vi "TLB Native Dynamic Events ver 0.26a.vi"() -> ()   [LabVIEW 2018] (continued)
      tunnel: w241 -> [w2776 w2788 w2804 w2825 w2838 w2853 w2867 w2881 w2897 w2912 w2925 w2937 w2953 w2971 w2992 w3008 w3025 w3036 w3063 w3079 w3090 w3103 w3118 w3131 w3146 w3171 w3207 w3233 w3247 w3258 w3270 w3286 w3302 w3315 w3326 w3351 w3374 w3386 w3396 w3407 w3420 w3433 w3446 w3461 w3472 w3489 w3503 w3517 w3532 w3547 w3562 w3577 w3592 w3606]
      tunnel: [w2776 w2788 w2804 w2825 w2838 w2853 w2867 w2881 w2897 w2912 w2925 w2937 w2953 w2971 w2992 w3008 w3025 w3036 w3062 w3079 w3090 w3103 w3118 w3131 w3146 w3170 w3206 w3233 w3247 w3258 w3270 w3286 w3302 w3315 w3326 w3351 w3374 w3386 w3396 w3407 w3420 w3433 w3446 w3461 w3472 w3489 w3502 w3517 w3532 w3547 w3562 w3577 w3592 w3606] -> w240
      tunnel: w238 -> [w2775 w2787 w2802 w2826 w2836 w2851 w2865 w2880 w2895 w2910 w2924 w2936 w2952 w2964 w2987 w3009 w3026 w3035 w3053 w3078 w3089 w3102 w3117 w3130 w3145 w3167 w3203 w3232 w3244 w3257 w3269 w3285 w3301 w3314 w3325 w3352 w3375 w3387 w3395 w3406 w3417 w3430 w3443 w3462 w3473 w3490 w3497 w3518 w3533 w3548 w3563 w3578 w3593 w3607]
      tunnel: [w2775 w2787 w2802 w2826 w2836 w2851 w2865 w2880 w2895 w2910 w2924 w2936 w2952 w2964 w2986 w3009 w3026 w3035 w3052 w3078 w3089 w3102 w3117 w3130 w3145 w3166 w3202 w3232 w3244 w3257 w3269 w3285 w3301 w3314 w3325 w3352 w3375 w3387 w3395 w3406 w3417 w3430 w3443 w3462 w3473 w3490 w3497 w3518 w3533 w3548 w3563 w3578 w3593 w3607] -> w237
      tunnel: w235 -> [w2773 w2786 w2803 w2827 w2837 w2852 w2866 w2879 w2896 w2911 w2923 w2935 w2951 w2963 w2983 w3010 w3027 w3034 w3049 w3075 w3088 w3101 w3116 w3129 w3144 w3164 w3200 w3230 w3243 w3256 w3268 w3284 w3300 w3313 w3324 w3353 w3376 w3388 w3394 w3405 w3416 w3429 w3442 w3463 w3474 w3491 w3496 w3512 w3527 w3542 w3557 w3572 w3587 w3601]
      tunnel: [w2773 w2786 w2803 w2827 w2837 w2852 w2866 w2879 w2896 w2911 w2923 w2935 w2951 w2963 w2983 w3010 w3027 w3034 w3049 w3075 w3088 w3101 w3116 w3129 w3143 w3163 w3199 w3230 w3243 w3256 w3268 w3284 w3300 w3313 w3324 w3353 w3376 w3388 w3394 w3405 w3416 w3429 w3442 w3463 w3474 w3491 w3496 w3512 w3525 w3540 w3555 w3570 w3585 w3600] -> w234
      tunnel: w232 -> [_ _ _ _ _ _ _ _ _ _ _ _ _ _ _ _ _ _ _ _ _ _ _ _ _ _ _ _ _ _ _ _ _ _ _ _ _ _ _ _ _ _ _ _ _ w3482 _ _ _ _ _ _ _ _]
      tunnel: [w2772 w2785 w2797 w2817 w2831 w2846 w2861 w2875 w2891 w2905 w2920 w2934 w2945 w2962 w2980 w3001 w3028 w3033 w3046 w3074 w3087 w3100 w3115 w3126 w3137 w3157 w3191 w3229 w3242 w3255 w3273 w3278 w3294 w3310 w3322 w3337 w3369 w3380 w3400 w3404 w3415 w3428 w3441 w3454 w3475 w3480 w3495 w3511 w3522 w3537 w3552 w3567 w3582 w3597] -> w228
      tunnel: w229 -> [w2772 w2785 w2797 w2817 w2831 w2846 w2861 w2875 w2891 w2905 w2920 w2934 w2945 w2962 w2980 w3002 w3028 w3033 w3046 w3074 w3087 w3100 w3115 w3126 w3137 w3158 w3192 w3229 w3242 w3255 w3273 w3278 w3294 w3310 w3322 w3337 w3369 w3380 w3400 w3404 w3415 w3428 w3441 w3454 w3475 w3480 w3495 w3511 w3522 w3537 w3552 w3567 w3582 w3597]
      tunnel: w226 -> [_ _ _ _ _ _ _ _ w2890 _ _ _ _ _ _ _ _ _ _ _ _ _ _ _ _ _ _ _ _ _ _ _ _ _ _ _ _ _ _ _ _ _ _ _ _ _ _ _ _ _ _ _ _ _]
      tunnel: w224 -> [w2771 w2784 w2796 w2811 w2830 w2845 w2860 w2874 w2888 w2904 w2919 w2933 w2944 w2961 w2979 w2997 w3021 w3032 w3044 w3073 w3086 w3099 w3114 w3125 w3140 w3160 w3195 w3228 w3241 w3254 w3265 w3277 w3293 w3309 w3321 w3334 w3368 w3379 w3391 w3403 w3414 w3427 w3440 w3453 w3466 w3479 w3494 w3510 w3521 w3536 w3551 w3566 w3581 w3596]
      tunnel: [w2771 w2784 w2796 w2811 w2830 w2845 w2860 w2874 w2888 w2904 w2919 w2933 w2944 w2961 w2979 w2997 w3020 w3032 w3044 w3073 w3086 w3099 w3114 w3125 w3139 w3159 w3194 w3228 w3241 w3254 w3265 w3277 w3293 w3309 w3321 w3334 w3368 w3379 w3391 w3403 w3414 w3427 w3440 w3453 w3466 w3479 w3494 w3510 w3521 w3536 w3551 w3566 w3581 w3596] -> w223
      tunnel: [_ _ _ _ _ _ _ _ _ _ _ _ _ _ _ _ _ _ _ _ _ _ _ _ _ _ _ _ _ _ _ _ _ _ _ w3333 w3363 _ _ _ _ _ _ _ _ _ _ _ _ _ _ _ _ _] -> w221
      tunnel: w219 -> [w2770 w2783 w2795 w2810 w2829 w2844 w2859 w2873 w2887 w2903 w2918 w2932 w2943 w2960 w2978 w2996 w3012 w3031 w3042 w3072 w3085 w3098 w3113 w3124 w3141 w3161 w3196 w3227 w3240 w3253 w3264 w3276 w3292 w3308 w3320 w3332 w3367 w3378 w3390 w3402 w3413 w3426 w3439 w3452 w3465 w3478 w3493 w3509 w3520 w3535 w3550 w3565 w3580 w3595]
      tunnel: [w2770 w2783 w2795 w2810 w2829 w2844 w2859 w2873 w2887 w2903 w2918 w2932 w2943 w2960 w2978 w2996 w3012 w3031 w3042 w3072 w3085 w3098 w3113 w3124 w3141 w3161 w3196 w3227 w3240 w3253 w3264 w3276 w3292 w3308 w3320 w3332 w3367 w3378 w3390 w3402 w3413 w3426 w3439 w3452 w3465 w3478 w3493 w3509 w3520 w3535 w3550 w3565 w3580 w3595] -> w218
      tunnel: w214 -> [w2769 w2782 w2794 w2809 w2828 w2843 w2858 w2872 w2886 w2902 w2917 w2931 w2942 w2959 w2977 w2993 w3011 w3030 w3041 w3071 w3084 w3097 w3112 w3123 w3136 w3154 w3189 w3226 w3239 w3252 w3263 w3275 w3291 w3307 w3319 w3331 w3361 w3377 w3389 w3401 w3412 w3425 w3438 w3451 w3464 w3477 w3492 w3508 w3519 w3534 w3549 w3564 w3579 w3594]
      tunnel: [w2769 w2782 w2794 w2809 w2828 w2843 w2858 w2872 w2886 w2902 w2917 w2931 w2942 w2959 w2977 w2993 w3011 w3030 w3041 w3071 w3084 w3097 w3112 w3123 w3136 w3154 w3189 w3226 w3239 w3252 w3263 w3275 w3291 w3307 w3319 w3331 w3354 w3377 w3389 w3401 w3412 w3425 w3438 w3451 w3464 w3477 w3492 w3508 w3519 w3534 w3549 w3564 w3579 w3594] -> w213
      frame "Exit" {
        # ">>State Logic  >>"
        # ">>> Time cluster >>>"
        # ">>> Yaw >>>"
        # ">>> Stepper position >>>"
        # ">>> Encoders >>>"
        # ">>> Object detection >>>"
        # ">>> Ultrasonic Sensors Detect >>>"
        n70 = call "Imaq Dispose"("All Images? (No)"=TRUE) -> ()  [unwired: 5 in, 1 out]
      }
      frame "----Movement States----" {
        # ">>State Logic  >>"
        # ">>> Time cluster >>>"
        # ">>> Yaw >>>"
        # ">>> Stepper position >>>"
        # ">>> Encoders >>>"
        # ">>> Object detection >>>"
        # ">>> Ultrasonic Sensors Detect >>>"
      }
      frame "FORWARD" {
        # ">>State Logic  >>"
        # ">>> Time cluster >>>"
        # ">>> Yaw >>>"
        # ">>> Stepper position >>>"
        # ">>> Encoders >>>"
        # ">>> Object detection >>>"
        # ">>> Ultrasonic Sensors Detect >>>"
        n71 = Unbundle By Name(w2802) -> ("Yaw"=w2798:dbl)
        n72 = call "MOTOR CONTROL WITH PID AE.vi"("Yaw"=w2798, "Speed"=50.0, "Direction"=MOTOR_CONTROL_WITH_PID_AE_DIRECTION_TYPE_DEF."y-axis movement", "AE Mode"=MOTOR_CONTROL_WITH_PID_AE_DATA_MODE_TYPE_DEF."Write to AE") -> ()  [unwired: 1 out]
      }
      frame "FORWARD - IR ASSIST" {
        # ">>State Logic  >>"
        # ">>> Time cluster >>>"
        # ">>> Yaw >>>"
        # ">>> Stepper position >>>"
        # ">>> Encoders >>>"
        # ">>> Object detection >>>"
        # ">>> Ultrasonic Sensors Detect >>>"
        n73 = Unbundle By Name(w2817) -> ("Left IR Sensor"=w2816:dbl)
        n74 = Subtract(x=w2816, y=15.0) -> (x-y=w2814:dbl)
        n75 = Multiply(x=w2814, y=0.25) -> (x*y=w2812:dbl)
        n76 = call "MOTOR CONTROL WITH PID AE.vi"("Yaw"=w2812, "Speed"=30.0, "Direction"=MOTOR_CONTROL_WITH_PID_AE_DIRECTION_TYPE_DEF."y-axis movement", "AE Mode"=MOTOR_CONTROL_WITH_PID_AE_DATA_MODE_TYPE_DEF."Write to AE") -> ()  [unwired: 1 out]
      }
      frame "LEFT" {
        # ">>State Logic  >>"
        # ">>> Time cluster >>>"
        # ">>> Yaw >>>"
        # ">>> Stepper position >>>"
        # ">>> Encoders >>>"
        # ">>> Object detection >>>"
        # ">>> Ultrasonic Sensors Detect >>>"
        n77 = Unbundle By Name(w2836) -> ("Yaw"=w2833:dbl)
        n78 = call "MOTOR CONTROL WITH PID AE.vi"("Yaw"=w2833, "Speed"=-20.0, "Direction"=MOTOR_CONTROL_WITH_PID_AE_DIRECTION_TYPE_DEF."x-axis movement", "AE Mode"=MOTOR_CONTROL_WITH_PID_AE_DATA_MODE_TYPE_DEF."Write to AE") -> ()  [unwired: 1 out]
      }
      frame "RIGHT" {
        # ">>> Time cluster >>>"
        # ">>> Yaw >>>"
        # ">>> Stepper position >>>"
        # ">>> Encoders >>>"
        # ">>> Object detection >>>"
        # ">>> Ultrasonic Sensors Detect >>>"
        n79 = Unbundle By Name(w2851) -> ("Yaw"=w2847:dbl)
        n80 = call "MOTOR CONTROL WITH PID AE.vi"("Yaw"=w2847, "Speed"=20.0, "Direction"=MOTOR_CONTROL_WITH_PID_AE_DIRECTION_TYPE_DEF."x-axis movement", "AE Mode"=MOTOR_CONTROL_WITH_PID_AE_DATA_MODE_TYPE_DEF."Write to AE") -> ()  [unwired: 1 out]
      }
      frame "R-ACW" {
        # ">>> IR Sensors >>>"
        # ">>> Time cluster >>>"
        # ">>> Yaw >>>"
        # ">>> Stepper position >>>"
        # ">>> Encoders >>>"
        # ">>> Object detection >>>"
        # ">>> Ultrasonic Sensors Detect >>>"
        n81 = call "MOTOR CONTROL WITH PID AE.vi"("Speed"=10.0, "Direction"=MOTOR_CONTROL_WITH_PID_AE_DIRECTION_TYPE_DEF."rotation", "AE Mode"=MOTOR_CONTROL_WITH_PID_AE_DATA_MODE_TYPE_DEF."Write to AE") -> ()  [unwired: 1 in, 1 out]
      }
      frame "R-CW" {
        (unwired) -0.2 ("Speed")
        # ">>> Time cluster >>>"
        # ">>> Yaw >>>"
        # ">>> Stepper position >>>"
        # ">>> Encoders >>>"
        # ">>> Object detection >>>"
        # ">>> Ultrasonic Sensors Detect >>>"
        n82 = call "MOTOR CONTROL WITH PID AE.vi"("Speed"=-10.0, "Direction"=MOTOR_CONTROL_WITH_PID_AE_DIRECTION_TYPE_DEF."rotation", "AE Mode"=MOTOR_CONTROL_WITH_PID_AE_DATA_MODE_TYPE_DEF."Write to AE") -> ()  [unwired: 1 in, 1 out]
      }
      frame "X AXIS - SLOW" {
        # ">>> Line Sensor Cluster>>>"
        # ">>> IR Sensors >>>"
        # ">>> Time cluster >>>"
        # ">>> Yaw >>>"
        # ">>> Stepper position >>>"
        # ">>> Encoders >>>"
        # ">>> Object detection >>>"
        # ">>> Ultrasonic Sensors Detect >>>"
        n83 = Unbundle By Name(w2890) -> ("xSpeed"=w2889:dbl)
        n84 = Unbundle By Name(w2895) -> ("Yaw"=w2892:dbl)
        n85 = call "MOTOR CONTROL WITH PID AE.vi"("Yaw"=w2892, "Speed"=w2889, "Direction"=MOTOR_CONTROL_WITH_PID_AE_DIRECTION_TYPE_DEF."x-axis movement", "AE Mode"=MOTOR_CONTROL_WITH_PID_AE_DATA_MODE_TYPE_DEF."Write to AE") -> ()  [unwired: 1 out]
      }
      frame "REVERSE" {
        # ">>> Time cluster >>>"
        # ">>> Yaw >>>"
        # ">>> Stepper position >>>"
        # ">>> Encoders >>>"
        # ">>> Object detection >>>"
        # ">>> Ultrasonic Sensors Detect >>>"
        n86 = Unbundle By Name(w2910) -> ("Yaw"=w2906:dbl)
        n87 = call "MOTOR CONTROL WITH PID AE.vi"("Yaw"=w2906, "Speed"=-50.0, "Direction"=MOTOR_CONTROL_WITH_PID_AE_DIRECTION_TYPE_DEF."y-axis movement", "AE Mode"=MOTOR_CONTROL_WITH_PID_AE_DATA_MODE_TYPE_DEF."Write to AE") -> ()  [unwired: 1 out]
      }
      frame "STOP" {
        n88 = Wait (ms)(milliseconds to wait=u32 100) -> ()  [unwired: 1 out]
        n89 = call "MOTOR CONTROL WITH PID AE.vi"("Direction"=MOTOR_CONTROL_WITH_PID_AE_DIRECTION_TYPE_DEF."stop", "AE Mode"=MOTOR_CONTROL_WITH_PID_AE_DATA_MODE_TYPE_DEF."Write to AE") -> ()  [unwired: 2 in, 1 out]
      }
      frame "----SENSOR READING---- " {
      }
      frame "READ ENCODERS" {
        # ">>> Time cluster >>>"
        # ">>> Yaw >>>"
        # ">>> Stepper position >>>"
        # ">>> Object detection >>>"
        # ">>> Current encoder distance >>>"
        # ">>> Ultrasonic Sensors Detect >>>"
        n90 = call "MOTOR CONTROL WITH PID AE.vi"("AE Mode"=MOTOR_CONTROL_WITH_PID_AE_DATA_MODE_TYPE_DEF."Read from AE") -> ("Speed & distance"=w2949:T15)  [unwired: 3 in]
        n91 = Unbundle By Name(w2949) -> ("xDistance"=w2948:dbl, "yDistance"=w2947:dbl, "wDistance"=w2946:dbl)
        n92 = Bundle By Name(cluster=w2956, "xDistance"=w2948, "yDistance"=w2947, "wDistance"=w2946) -> (w2955:T8)
      }
      frame "READ ULTRASONIC" {
        (unwired) navX_type_def."Read Values" ("Mode")
        (unwired) MOTOR_CONTROL_NO_PID_Type_Def."Latch" ("Direction")
        # ">>> Line Sensor Cluster>>>"
        # ">>> IR Sensors >>>"
        # ">>State Logic  >>"
        # ">>> Time cluster >>>"
        # ">>> Ultrasonic Sensors Detect >>>"
        # ">>> Object detection >>>"
        # ">>> Encoders >>>"
        # ">>> Stepper position >>>"
        # ">>> Yaw >>>"
        n93 = call "Arduino Interfacing VI.vi"("AE Mode"=Arduino_Interfacing."Read From Arduino") -> ("Arduino Data"=w2969:T17)  [unwired: 3 in, 1 out]
        n94 = Unbundle By Name(w2969) -> ("PING A"=w2968:u8, "PING B"=w2967:u8, "PING C"=w2966:u8, "PING D"=w2965:u8)
        n95 = Bundle By Name(cluster=w2975, "PING_A"=w2968, "PING_B"=w2967, "PING_C"=w2966, "PING_D"=w2965) -> (w2976:T9)
      }
      frame "READ NAVX" {
        # ">> Item Selection Bias >>"
        # ">>State Logic  >>"
        # ">>> Line Sensor Cluster>>>"
        # ">>> IR Sensors >>>"
        # ">>> Time cluster >>>"
        # ">>> Yaw >>>"
        # ">>> Ultrasonic Sensors Detect >>>"
        # ">>> Object detection >>>"
        # ">>> Encoders >>>"
        # ">>> Stepper position >>>"
        n96 = call "navX reading VI.vi"("Mode"=navX_type_def."Read Values") -> ("NavX Readings"=w2982:T16)  [unwired: 2 in, 3 out]
        n97 = Unbundle By Name(w2982) -> ("Heading"=w2981:dbl)
        n98 = Unbundle By Name(w2982) -> ("Yaw"=w2985:dbl)
        n99 = Bundle By Name(cluster=w2987, "Yaw"=w2985, "Compass"=w2981) -> (w2986:T6)
      }
      frame "READ IR" {
        w2995 = T41 [enum."B/AI2"] items=["Not Connected", "AudioIn/Left", "AudioIn/Right", "C/AI0", "C/AI1", "A/AI0", "A/AI1", "A/AI2", "A/AI3", "A/AI4", "A/AI5", "A/AI6", "A/AI7", "B/AI0", "B/AI1", "B/AI2", "B/AI3", "B/AI4", "B/AI5", "B/AI6", "B/AI7", "AI/AI0", "AI/AI1", "AI/AI2", "AI/AI3", "A/AI0 (DIFF)", "A/AI1 (DIFF)", "A/AI2 (DIFF)", "A/AI3 (DIFF)", "B/AI0 (DIFF)", "B/AI1 (DIFF)", "B/AI2 (DIFF)", "B/AI3 (DIFF)"] ("AI Channel")
        w2999 = T41 [enum."B/AI1"] items=["Not Connected", "AudioIn/Left", "AudioIn/Right", "C/AI0", "C/AI1", "A/AI0", "A/AI1", "A/AI2", "A/AI3", "A/AI4", "A/AI5", "A/AI6", "A/AI7", "B/AI0", "B/AI1", "B/AI2", "B/AI3", "B/AI4", "B/AI5", "B/AI6", "B/AI7", "AI/AI0", "AI/AI1", "AI/AI2", "AI/AI3", "A/AI0 (DIFF)", "A/AI1 (DIFF)", "A/AI2 (DIFF)", "A/AI3 (DIFF)", "B/AI0 (DIFF)", "B/AI1 (DIFF)", "B/AI2 (DIFF)", "B/AI3 (DIFF)"] ("AI Channel")
        w3004 = T41 [enum."B/AI0"] items=["Not Connected", "AudioIn/Left", "AudioIn/Right", "C/AI0", "C/AI1", "A/AI0", "A/AI1", "A/AI2", "A/AI3", "A/AI4", "A/AI5", "A/AI6", "A/AI7", "B/AI0", "B/AI1", "B/AI2", "B/AI3", "B/AI4", "B/AI5", "B/AI6", "B/AI7", "AI/AI0", "AI/AI1", "AI/AI2", "AI/AI3", "A/AI0 (DIFF)", "A/AI1 (DIFF)", "A/AI2 (DIFF)", "A/AI3 (DIFF)", "B/AI0 (DIFF)", "B/AI1 (DIFF)", "B/AI2 (DIFF)", "B/AI3 (DIFF)"] ("AI Channel")
        # ">>> Line Sensor Cluster>>>"
        # ">>> IR Sensors >>>"
        # ">>State Logic  >>"
        # ">>> Time cluster >>>"
        # ">>> Ultrasonic Sensors Detect >>>"
        # ">>> Object detection >>>"
        # ">>> Encoders >>>"
        # ">>> Stepper position >>>"
        # ">>> Yaw >>>"
        n100 = call <vilib>:"Sharp IR.vi"("AI Channel"=w3004) -> ("Sharp IR Distance"=w3000:dbl)  [unwired: 8 in, 2 out]
        n101 = call <vilib>:"Sharp IR.vi"("AI Channel"=w2999) -> ("Sharp IR Distance"=w2998:dbl)  [unwired: 8 in, 2 out]
        n102 = call <vilib>:"Sharp IR.vi"("AI Channel"=w2995) -> ("Sharp IR Distance"=w2994:dbl)  [unwired: 8 in, 2 out]
        n103 = Bundle By Name(cluster=w3002, "Left IR Sensor"=w3000, "Arm IR Sensor"=w2998, "Bottom IR Sensor"=w2994) -> (w3001:T5)
      }
      frame "READ LINE SENSOR" {
        # ">>> IR Sensors >>>"
        # ">>> Line Sensor Cluster>>>"
        # ">>State Logic  >>"
        # ">>> Time cluster >>>"
        # ">>> Object detection >>>"
        # ">>> Yaw >>>"
        # ">>> Ultrasonic Sensors Detect >>>"
        # ">>> Encoders >>>"
        # ">>> Stepper position >>>"
        n104 = call "Line Sensor AE.vi"("AE State"=Line_Sensor_AE_Type_Def."READ FROM LINE SENSORS") -> ("Line Detected?"=w3018:bool, "Line Sensor Raw Values"=w3017:T43)
        n105 = Unbundle By Name(w3017) -> ("S1"=w3016:dbl, "S2"=w3015:dbl, "S3"=w3014:dbl, "S4"=w3013:dbl)
        n106 = Bundle By Name(cluster=w3021, "Line Detected?"=w3018, "S1"=w3016, "S2"=w3015, "S3"=w3014, "S4"=w3013) -> (w3020:T4)
      }
      frame "----SYSTEM MODES----" {
        (unwired) I2C_MASTER_Type_Def."Last State" ("Arduino Mode")
        # ">>> Object detection >>>"
        # ">>> Yaw >>>"
        # ">>> Ultrasonic Sensors Detect >>>"
        # ">>> Encoders >>>"
        # ">>> Stepper position >>>"
      }
      frame "INIT" {
        w3064 = u8 0
        w3065 = 0.0
        # ">>> IR Sensors >>>"
        # ">>> IR Sensors >>>"
        # ">>> Line Sensor Cluster>>>"
        # ">>> Time cluster >>>"
        # ">>> Object detection >>>"
        # ">>> Yaw >>>"
        # ">>> Ultrasonic Sensors Detect >>>"
        # ">>> Encoders >>>"
        # ">>> Stepper position >>>"
        # ">>State Logic  >>"
        n107 = call "Arduino Interfacing VI.vi"("AE Mode"=Arduino_Interfacing."Initialize") -> ()  [unwired: 3 in, 2 out]
        n108 = call "FGV Stop.vi"("Init/Read/Write State"=States_for_Action_Engine."Initialize") -> ()  [unwired: 2 in, 2 out]
        n109 = call "Elasped Timer.vi"("Action"=Elapsed_timer_control."Initialize") -> ()  [unwired: 7 in, 4 out]
        n110 = call "MOTOR CONTROL WITH PID AE.vi"("AE Mode"=MOTOR_CONTROL_WITH_PID_AE_DATA_MODE_TYPE_DEF."Init AE") -> ()  [unwired: 3 in, 1 out]
        n111 = call "IMAQ Reference AE.vi"("IMAQ AE States"=IMAQ_Reference_AE."Initialize AE") -> ()  [unwired: 1 in, 2 out]
        n112 = call "Line Sensor AE.vi"("AE State"=Line_Sensor_AE_Type_Def."INIT AE") -> ()  [unwired: 2 out]
        n113 = Bundle By Name(cluster=w3058, "Recognized Object"=FALSE, "Object X coordinate"=0.0, "Object Y coordinate"=0.0) -> (w3057:T11)
        n114 = Bundle By Name(cluster=w3063, "y Stepper Position"=u8 0, "z Stepper Position"=u8 0) -> (w3062:T7)
        n115 = Bundle By Name(cluster=w3067, "xDistance"=w3065, "yDistance"=w3065, "wDistance"=w3065) -> (w3066:T8)
        n116 = Bundle By Name(cluster=w3069, "PING_A"=w3064, "PING_B"=w3064, "PING_C"=w3064, "PING_D"=w3064) -> (w3070:T9)
        n117 = Bundle By Name(cluster=w3053, "Yaw"=0.0) -> (w3052:T6)
      }
      frame "ARDUINO - ULTRASONIC" {
        # ">>> Time cluster >>>"
        # ">>> Line Sensor Cluster>>>"
        # ">>> Object detection >>>"
        # ">>> Yaw >>>"
        # ">>> Ultrasonic Sensors Detect >>>"
        # ">>> Encoders >>>"
        # ">>> Stepper position >>>"
        # ">>State Logic  >>"
        n118 = call "Arduino Interfacing VI.vi"("Data to Write"=I2C_MASTER_WRITE_NEW_Type_Def."Ultrasonic sensors", "AE Mode"=Arduino_Interfacing."Write to Arduino") -> ()  [unwired: 2 in, 2 out]
      }
      frame "NAVX CALIBRATE" {
        # ">>> Object detection >>>"
        # ">>> Yaw >>>"
        # ">>> Ultrasonic Sensors Detect >>>"
        # ">>> Encoders >>>"
        # ">>> Stepper position >>>"
        # ">>State Logic  >>"
        # "Adds a 15 second delay to the startup process \nfor the NavX to calibrate"
        n119 = Wait (ms)(milliseconds to wait=u32 1000) -> ()  [unwired: 1 out]
      }
      frame "NO ACTION", Default {
        (unwired) u8 0 ("y Stepper value")
        (unwired) TRUE ("Latch")
        (unwired) navX_type_def."Read Values" ("Mode")
        (unwired) MOTOR_CONTROL_NO_PID_Type_Def."Latch" ("Direction")
        # ">>> Object detection >>>"
        # ">>> Yaw >>>"
        # ">>> Ultrasonic Sensors Detect >>>"
        # ">>> Encoders >>>"
        # ">>> Stepper position >>>"
        # ">>State Logic  >>"
        n120 = case shown="4" w3106 {
          tunnel: [0 100] -> w3108
          frame 1, Default {
          }
          frame 4 {
          }
        }
      }
      frame "----RESET CASES----" {
        (unwired) I2C_MASTER_Type_Def."Last State" ("Arduino Mode")
        # ">>> Object detection >>>"
        # ">>> Yaw >>>"
        # ">>> Ultrasonic Sensors Detect >>>"
        # ">>> Encoders >>>"
        # ">>> Stepper position >>>"
        # ">>State Logic  >>"
      }
      frame "RESET ENCODERS" {
        # ">>> Object detection >>>"
        # ">>> Yaw >>>"
        # ">>> Ultrasonic Sensors Detect >>>"
        # ">>> Encoders >>>"
        # ">>> Stepper position >>>"
        # ">>State Logic  >>"
        n121 = call "MOTOR CONTROL WITH PID AE.vi"("Direction"=MOTOR_CONTROL_WITH_PID_AE_DIRECTION_TYPE_DEF."reset encoders", "AE Mode"=MOTOR_CONTROL_WITH_PID_AE_DATA_MODE_TYPE_DEF."Write to AE") -> ()  [unwired: 2 in, 1 out]
      }
      frame "RESET FLAGS" {
        # ">>> Line Sensor Cluster>>>"
        # ">>> IR Sensors >>>"
        # ">>> Time cluster >>>"
        # ">>> Object detection >>>"
        # ">>> Yaw >>>"
        # ">>> Ultrasonic Sensors Detect >>>"
        # ">>> Encoders >>>"
        # ">>> Stepper position >>>"
        # ">>> Line Sensor Cluster>>>"
        # ">>> IR Sensors >>>"
        # ">>> Time cluster >>>"
        # ">>> Object detection >>>"
        # ">>> Yaw >>>"
        # ">>> Ultrasonic Sensors Detect >>>"
        # ">>> Encoders >>>"
        # ">>> Stepper position >>>"
        # "Resets BOOLEAN FLAGS only"
        n122 = Wait (ms)(milliseconds to wait=u32 20) -> ()  [unwired: 1 out]
        n123 = Bundle By Name(cluster=w3150, "Recognized Object"=FALSE) -> (w3149:T11)
        n124 = Bundle By Name(cluster=w3140, "Line Detected?"=FALSE) -> (w3139:T4)
        n125 = Bundle By Name(cluster=w3144, "Time up flag"=FALSE) -> (w3143:T3)
      }
      frame "RESET SENSOR VALUES" {
        w3155 = 0.0 ("S4")
        w3156 = 0.0 ("S4")
        # "Resets SENSOR VALUES only"
        # ">>> Line Sensor Cluster>>>"
        # ">>> IR Sensors >>>"
        # ">>> Time cluster >>>"
        # ">>> Object detection >>>"
        # ">>> Yaw >>>"
        # ">>> Ultrasonic Sensors Detect >>>"
        # ">>> Encoders >>>"
        # ">>> Stepper position >>>"
        # ">>> Line Sensor Cluster>>>"
        # ">>> IR Sensors >>>"
        # ">>> Time cluster >>>"
        # ">>> Object detection >>>"
        # ">>> Yaw >>>"
        # ">>> Ultrasonic Sensors Detect >>>"
        # ">>> Encoders >>>"
        # ">>> Stepper position >>>"
        # "Resets any software variables\nand/or non-critical states"
        n126 = Wait (ms)(milliseconds to wait=u32 20) -> ()  [unwired: 1 out]
        n127 = Bundle By Name(cluster=w3164, "SET TIME TO CHECK"=0.0) -> (w3163:T3)
        n128 = Bundle By Name(cluster=w3180, "Object X coordinate"=0.0, "Object Y coordinate"=0.0) -> (w3179:T11)
        n129 = Bundle By Name(cluster=w3171, "y Stepper Position"=u8 0, "z Stepper Position"=u8 0) -> (w3170:T7)
        n130 = Bundle By Name(cluster=w3158, "Left IR Sensor"=w3155, "Arm IR Sensor"=w3155) -> (w3157:T5)
        n131 = Bundle By Name(cluster=w3176, "xDistance"=0.0, "yDistance"=0.0, "wDistance"=0.0) -> (w3175:T8)
        n132 = Bundle By Name(cluster=w3187, "PING_A"=u8 0, "PING_B"=u8 0, "PING_C"=u8 0, "PING_D"=u8 0) -> (w3186:T9)
        n133 = Bundle By Name(cluster=w3167, "Yaw"=0.0) -> (w3166:T6)
        n134 = Bundle By Name(cluster=w3160, "S1"=w3156, "S2"=w3156, "S3"=w3156, "S4"=w3156) -> (w3159:T4)
      }
      frame "RESET ALL SENSORS" {
        w3190 = 0.0 ("SET TIME TO CHECK")
        # ">>> Line Sensor Cluster>>>"
        # ">>> IR Sensors >>>"
        # ">>> Time cluster >>>"
        # ">>> Object detection >>>"
        # ">>> Yaw >>>"
        # ">>> Ultrasonic Sensors Detect >>>"
        # ">>> Encoders >>>"
        # ">>> Stepper position >>>"
        # ">>> Line Sensor Cluster>>>"
        # ">>> IR Sensors >>>"
        # ">>> Time cluster >>>"
        # ">>> Object detection >>>"
        # ">>> Yaw >>>"
        # ">>> Ultrasonic Sensors Detect >>>"
        # ">>> Encoders >>>"
        # ">>> Stepper position >>>"
        # "Resets ALL SENSOR PARAMTERS"
        n135 = Wait (ms)(milliseconds to wait=u32 20) -> ()  [unwired: 1 out]
        n136 = Bundle By Name(cluster=w3200, "Time up flag"=FALSE, "SET TIME TO CHECK"=0.0) -> (w3199:T3)
        n137 = Bundle By Name(cluster=w3217, "Recognized Object"=FALSE, "Object X coordinate"=0.0, "Object Y coordinate"=0.0) -> (w3216:T11)
        n138 = Bundle By Name(cluster=w3207, "y Stepper Position"=u8 0, "z Stepper Position"=u8 0) -> (w3206:T7)
        n139 = Bundle By Name(cluster=w3195, "Line Detected?"=FALSE) -> (w3194:T4)
        n140 = Bundle By Name(cluster=w3192, "Left IR Sensor"=w3190, "Arm IR Sensor"=w3190) -> (w3191:T5)
        n141 = Bundle By Name(cluster=w3212, "xDistance"=0.0, "yDistance"=0.0, "wDistance"=0.0) -> (w3211:T8)
        n142 = Bundle By Name(cluster=w3224, "PING_A"=u8 0, "PING_B"=u8 0, "PING_C"=u8 0, "PING_D"=u8 0) -> (w3223:T9)
        n143 = Bundle By Name(cluster=w3203, "Yaw"=0.0) -> (w3202:T6)
      }
      frame "RESET YAW" {
        n144 = Wait (ms)(milliseconds to wait=u32 100) -> ()  [unwired: 1 out]
        n145 = call "navX reading VI.vi"("Mode"=navX_type_def."Zero Yaw") -> ()  [unwired: 2 in, 4 out]
      }
      frame "RESET ARM" {
        n146 = call "Arduino Interfacing VI.vi"("Data to Write"=I2C_MASTER_WRITE_NEW_Type_Def."Soft Reset", "AE Mode"=Arduino_Interfacing."Write to Arduino") -> ()  [unwired: 2 in, 2 out]
      }
      frame "--------CAM STATES-------" {
      }
      frame "OPEN IMAQ REF" {
        # ">>> Line Sensor Cluster>>>"
        # ">>State Logic  >>"
        # ">>> Time cluster >>>"
        # ">>> Object detection >>>"
        # ">>> Yaw >>>"
        # ">>> Ultrasonic Sensors Detect >>>"
        # ">>> Encoders >>>"
        # ">>> Stepper position >>>"
        # ">>> IR Sensors >>>"
        n147 = call "IMAQ Reference AE.vi"("IMAQ AE States"=IMAQ_Reference_AE."Initialize AE") -> ()  [unwired: 1 in, 2 out]
      }
      frame "OPEN LOG CAM" {
        n148 = call "Webcam AE.vi"("Session In"=T39 "cam0", "Camera states"=Webcam_AE."Initialize Camera") -> ("error out"=w3281:errorcluster, "Session Out"=w3280:T39)  [unwired: 1 in, 1 out]
        n149 = call "Webcam AE.vi"("error in (no error)"=w3281, "Session In"=w3280, "Camera states"=Webcam_AE."Open Camera") -> ()  [unwired: 3 out]
      }
      frame "OPEN LIFE CAM" {
        n150 = call "Webcam AE.vi"("Session In"=T39 "cam1", "Camera states"=Webcam_AE."Initialize Camera") -> ("error out"=w3297:errorcluster, "Session Out"=w3296:T39)  [unwired: 1 in, 1 out]
        n151 = call "Webcam AE.vi"("error in (no error)"=w3297, "Session In"=w3296, "Camera states"=Webcam_AE."Open Camera") -> ()  [unwired: 3 out]
      }
      frame "CAM ACQ" {
        # ">>State Logic  >>"
        # ">>> Time cluster >>>"
        # ">>> Yaw >>>"
        # ">>> Stepper position >>>"
        # ">>> Encoders >>>"
        # ">>> Object detection >>>"
        # ">>> Ultrasonic Sensors Detect >>>"
        n152 = call "Webcam AE.vi"("Camera states"=Webcam_AE."Continuous Acquisition") -> ()  [unwired: 2 in, 3 out]
      }
      frame "CAM CLOSE" {
        # ">>State Logic  >>"
        # ">>> Time cluster >>>"
        # ">>> Yaw >>>"
        # ">>> Stepper position >>>"
        # ">>> Encoders >>>"
        # ">>> Object detection >>>"
        # ">>> Ultrasonic Sensors Detect >>>"
        n153 = call "Webcam AE.vi"("Camera states"=Webcam_AE."Close Camera") -> ()  [unwired: 2 in, 3 out]
      }
      frame "PROCESS IMAGE" {
        # ">>> Line Sensor Cluster>>>"
        # ">>> IR Sensors >>>"
        # ">> Item Selection Bias >>"
        # ">> Item Selection Bias >>"
        # ">>State Logic  >>"
        # ">>> Time cluster >>>"
        # ">>> Yaw >>>"
        # ">>> Stepper position >>>"
        # ">>> Encoders >>>"
        # ">>> Object detection >>>"
        # ">>> Ultrasonic Sensors Detect >>>"
        n154 = call "Webcam AE.vi"("Camera states"=Webcam_AE."Retrieve Image") -> ("error out"=w3345:errorcluster, "Image Out"=w3346:T45)  [unwired: 2 in, 1 out]
        n155 = call "IMAQ Reference AE.vi"("IMAQ AE States"=IMAQ_Reference_AE."Get IMAQ Reference") -> ("Image Out"=w3335:T45)  [unwired: 1 in, 1 out]
        n156 = call "Object Detection SubVI.vi"("Error In"=w3345, "Mode"=w3332, "Image Dest"=w3335, "Image in"=w3346) -> ("Error out"=w3333:errorcluster, "Object Center Coordinates"=w3342:cluster{"x":sgl, "y":sgl}, "Object detection cluster"=w3338:T46)  [unwired: 1 out]
        n157 = Unbundle By Name(w3338) -> ("Object detected?"=w3339:bool)
        n158 = Unbundle By Name(w3342) -> ("x"=w3341:sgl, "y"=w3340:sgl)
        n159 = Bundle By Name(cluster=w3344, "Recognized Object"=w3339, "Object X coordinate"=w3341, "Object Y coordinate"=w3340) -> (w3343:T11)
      }
      frame "COLOUR PROCESSING" {
        # ">>> Box Colour Detection >>>"
        # ">>> Box Colour Detection >>>"
        # ">>> Line Sensor Cluster>>>"
        # ">>> IR Sensors >>>"
        # ">> Item Selection Bias >>"
        # ">> Item Selection Bias >>"
        # ">>State Logic  >>"
        # ">>> Time cluster >>>"
        # ">>> Yaw >>>"
        # ">>> Stepper position >>>"
        # ">>> Encoders >>>"
        # ">>> Object detection >>>"
        # ">>> Ultrasonic Sensors Detect >>>"
        n160 = call "Webcam AE.vi"("Camera states"=Webcam_AE."Retrieve Image") -> ("error out"=w3364:errorcluster, "Image Out"=w3365:T45)  [unwired: 2 in, 1 out]
        n161 = call "Box Colour Detection SubVI.vi"("Image In"=w3365, "Error In"=w3364) -> ("Colour output boolean cluster"=w3362:T47, "Error out"=w3363:errorcluster)  [unwired: 1 out]
        n162 = Unbundle By Name(w3362) -> ("Red"=w3360:bool, "Black"=w3359:bool, "Blue"=w3358:bool, "Yellow"=w3357:bool, "Green"=w3356:bool, "No recognizable coolour"=w3355:bool)
        n163 = Bundle By Name(cluster=w3361, "Red"=w3360, "Black"=w3359, "Blue"=w3358, "Yellow"=w3357, "Green"=w3356, "Unknown"=w3355) -> (w3354:T1)
      }
      frame "DISPOSE CAM BUFFERS" {
        # ">> Item Selection Bias >>"
        # ">>> Line Sensor Cluster>>>"
        # ">>> IR Sensors >>>"
        # ">>State Logic  >>"
        # ">>> Time cluster >>>"
        # ">>> Yaw >>>"
        # ">>> Stepper position >>>"
        # ">>> Encoders >>>"
        # ">>> Object detection >>>"
        # ">>> Ultrasonic Sensors Detect >>>"
        n164 = call "Webcam AE.vi"("Camera states"=Webcam_AE."Dispose Camera Image Buffer") -> ()  [unwired: 2 in, 3 out]
      }
      frame "DISPOSE PROC BUFFERS" {
        # ">>> Line Sensor Cluster>>>"
        # ">>State Logic  >>"
        # ">>> IR Sensors >>>"
        # ">>> Time cluster >>>"
        # ">>> Object detection >>>"
        # ">>> Yaw >>>"
        # ">>> Ultrasonic Sensors Detect >>>"
        # ">>> Encoders >>>"
        # ">>> Stepper position >>>"
        n165 = call "IMAQ Reference AE.vi"("IMAQ AE States"=IMAQ_Reference_AE."Dispose Processing Buffer") -> ()  [unwired: 1 in, 2 out]
      }
      frame "-----ARM ACTIONS-----" {
      }
      frame "CLOSE CLAW" {
        n166 = call "Arduino Interfacing VI.vi"("Data to Write"=I2C_MASTER_WRITE_NEW_Type_Def."Close Claw", "AE Mode"=Arduino_Interfacing."Write to Arduino") -> ()  [unwired: 2 in, 2 out]
      }
      frame "OPEN CLAW" {
        n167 = call "Arduino Interfacing VI.vi"("Data to Write"=I2C_MASTER_WRITE_NEW_Type_Def."Open Claw", "AE Mode"=Arduino_Interfacing."Write to Arduino") -> ()  [unwired: 2 in, 2 out]
      }
      frame "Z STEPPER CAM HEIGHT" {
        n168 = call "Arduino Interfacing VI.vi"("Data to Write"=I2C_MASTER_WRITE_NEW_Type_Def."zStepper 6k", "AE Mode"=Arduino_Interfacing."Write to Arduino") -> ()  [unwired: 2 in, 2 out]
      }
      frame "Z STEPPER GRAB HEIGHT" {
        # ">>State Logic  >>"
        # ">>> Time cluster >>>"
        # ">>> Yaw >>>"
        # ">>> Stepper position >>>"
        # ">>> Encoders >>>"
        # ">>> Object detection >>>"
        # ">>> Ultrasonic Sensors Detect >>>"
        n169 = call "Arduino Interfacing VI.vi"("Data to Write"=I2C_MASTER_WRITE_NEW_Type_Def."zStepper 100", "AE Mode"=Arduino_Interfacing."Write to Arduino") -> ()  [unwired: 2 in, 2 out]
      }
      frame "Z STEPPER BOX HEIGHT" {
        # ">>> IR Sensors >>>"
        # ">>> Time cluster >>>"
        # ">>> Yaw >>>"
        # ">>> Stepper position >>>"
        # ">>> Encoders >>>"
        # ">>> Object detection >>>"
        # ">>> Ultrasonic Sensors Detect >>>"
        n170 = call "Arduino Interfacing VI.vi"("Data to Write"=I2C_MASTER_WRITE_NEW_Type_Def."zStepper 5k", "AE Mode"=Arduino_Interfacing."Write to Arduino") -> ()  [unwired: 2 in, 2 out]
      }
      frame "Y STEPPER CONTROL" {
        # ">>State Logic  >>"
        # ">>> yStepper command>>>"
        # ">>> Time cluster >>>"
        # ">>> Yaw >>>"
        # ">>> Stepper position >>>"
        # ">>> Encoders >>>"
        # ">>> Object detection >>>"
        # ">>> Ultrasonic Sensors Detect >>>"
        n171 = Unbundle By Name(w3482) -> ("yStepper desired"=w3481:u8)
        n172 = call "Arduino Interfacing VI.vi"("y Stepper value"=w3481, "Data to Write"=I2C_MASTER_WRITE_NEW_Type_Def."yStepper control", "AE Mode"=Arduino_Interfacing."Write to Arduino") -> ()  [unwired: 1 in, 2 out]
      }
      frame "READ STEPPER VALUES" {
        # ">>State Logic  >>"
        # ">>> Time cluster >>>"
        # ">>> Yaw >>>"
        # ">>> Stepper position >>>"
        # ">>> Encoders >>>"
        # ">>> Object detection >>>"
        # ">>> Ultrasonic Sensors Detect >>>"
        n173 = call "Arduino Interfacing VI.vi"("AE Mode"=Arduino_Interfacing."Read From Arduino") -> ("Arduino Data"=w3500:T17)  [unwired: 3 in, 1 out]
        n174 = Unbundle By Name(w3500) -> ("y Stepper Position"=w3499:u8, "z Stepper Position"=w3498:u8)
        n175 = Bundle By Name(cluster=w3503, "y Stepper Position"=w3499, "z Stepper Position"=w3498) -> (w3502:T7)
      }
      frame " -----TIMING-----" {
        # ">>State Logic  >>"
        # ">>> Time cluster >>>"
        # ">>> Yaw >>>"
        # ">>> Stepper position >>>"
        # ">>> Encoders >>>"
        # ">>> Object detection >>>"
        # ">>> Ultrasonic Sensors Detect >>>"
      }
      frame "SET TIMER 1" {
        # ">>State Logic  >>"
        # ">>> Time cluster >>>"
        # ">>> Yaw >>>"
        # ">>> Stepper position >>>"
        # ">>> Encoders >>>"
        # ">>> Object detection >>>"
        # ">>> Ultrasonic Sensors Detect >>>"
        n176 = call "Elasped Timer.vi"("Time Setting"=1.0, "Action"=Elapsed_timer_control."Initialize") -> ()  [unwired: 6 in, 4 out]
        n177 = Bundle By Name(cluster=w3527, "Time up flag"=FALSE) -> (w3525:T3)
      }
      frame "SET TIMER 2" {
        # ">>State Logic  >>"
        # ">>> Time cluster >>>"
        # ">>> Yaw >>>"
        # ">>> Stepper position >>>"
        # ">>> Encoders >>>"
        # ">>> Object detection >>>"
        # ">>> Ultrasonic Sensors Detect >>>"
        n178 = call "Elasped Timer.vi"("Time Setting"=2.0, "Action"=Elapsed_timer_control."Initialize") -> ()  [unwired: 6 in, 4 out]
        n179 = Bundle By Name(cluster=w3542, "Time up flag"=FALSE) -> (w3540:T3)
      }
      frame "SET TIMER 3" {
        # ">>State Logic  >>"
        # ">>> Time cluster >>>"
        # ">>> Yaw >>>"
        # ">>> Stepper position >>>"
        # ">>> Encoders >>>"
        # ">>> Object detection >>>"
        # ">>> Ultrasonic Sensors Detect >>>"
        n180 = call "Elasped Timer.vi"("Time Setting"=3.0, "Action"=Elapsed_timer_control."Initialize") -> ()  [unwired: 6 in, 4 out]
        n181 = Bundle By Name(cluster=w3557, "Time up flag"=FALSE) -> (w3555:T3)
      }
      frame "SET TIMER 4" {
        # ">>State Logic  >>"
        # ">>> Time cluster >>>"
        # ">>> Yaw >>>"
        # ">>> Stepper position >>>"
        # ">>> Encoders >>>"
        # ">>> Object detection >>>"
        # ">>> Ultrasonic Sensors Detect >>>"
        n182 = call "Elasped Timer.vi"("Time Setting"=4.0, "Action"=Elapsed_timer_control."Initialize") -> ()  [unwired: 6 in, 4 out]
        n183 = Bundle By Name(cluster=w3572, "Time up flag"=FALSE) -> (w3570:T3)
      }
      frame "SET TIMER 5" {
        # ">>State Logic  >>"
        # ">>> Time cluster >>>"
        # ">>> Yaw >>>"
        # ">>> Stepper position >>>"
        # ">>> Encoders >>>"
        # ">>> Object detection >>>"
        # ">>> Ultrasonic Sensors Detect >>>"
        n184 = call "Elasped Timer.vi"("Time Setting"=5.0, "Action"=Elapsed_timer_control."Initialize") -> ()  [unwired: 6 in, 4 out]
        n185 = Bundle By Name(cluster=w3587, "Time up flag"=FALSE) -> (w3585:T3)
      }
      frame "START TIMER" {
        # ">>State Logic  >>"
        # ">>> Time cluster >>>"
        # ">>> Yaw >>>"
        # ">>> Stepper position >>>"
        # ">>> Encoders >>>"
        # ">>> Object detection >>>"
        # ">>> Ultrasonic Sensors Detect >>>"
        n186 = call "Elasped Timer.vi"("Action"=Elapsed_timer_control."Start") -> ("Time Out?!"=w3598:bool)  [unwired: 7 in, 3 out]
        n187 = Bundle By Name(cluster=w3601, "Time up flag"=w3598) -> (w3600:T3)
      }
    }
    "State Logic" <- w254
    "Image Processing Error" <- w221
    n188 = local read "TASK ENABLE"() -> (w248:bool)
    n189 = Not(x=w248) -> (.not. x?=w247:bool)
    n190 = case shown="True" w255 {
      tunnel: w212 -> [w286 w331]
      tunnel: w262 -> [w282 w333]
      tunnel: [w286 w331] -> w267
      tunnel: [w282 w334] -> w266
      tunnel: w263 -> [_ w329]
      tunnel: w265 -> [_ w330]
      tunnel: w260 -> [w285 w336]
      tunnel: [w285 w336] -> w259
      tunnel: "STOP TASK" -> [_ w319]
      tunnel: w254 -> [w284 w335]
      tunnel: [w284 w332] -> w253
      tunnel: w250 -> [w283 w325]
      tunnel: [w283 w325] -> w249
      tunnel: w247 -> [_ w320]
      tunnel: [w281 w317] -> w246
      tunnel: w245 -> [w281 w316]
      tunnel: w243 -> [w280 w313]
      tunnel: [w280 w313] -> w242
      tunnel: w240 -> [w279 w309]
      tunnel: [w279 w309] -> w239
      tunnel: w237 -> [w278 w307]
      tunnel: [w278 w307] -> w236
      tunnel: w234 -> [w277 w305]
      tunnel: [w277 w305] -> w233
      tunnel: w232 -> [w276 w304]
      tunnel: [w276 w303] -> w231
      tunnel: [_ w301] -> w230
      tunnel: w228 -> [w275 w299]
      tunnel: [w275 w299] -> w227
      tunnel: w226 -> [w274 w298]
      tunnel: [w274 w297] -> w225
      tunnel: w223 -> [w273 w294]
      tunnel: [w273 w294] -> w222
      tunnel: [w272 w293] -> w220
      tunnel: w218 -> [w272 w292]
      tunnel: [_ w290] -> w217
      tunnel: [_ w289] -> w216
      tunnel: [_ w288] -> w215
      tunnel: w213 -> [w271 w287]
      tunnel: [w271 w287] -> w211
      frame False {
        # ">>> Box Colour Detection >>>"
        # ">>> Line Sensor Cluster>>>"
        # ">> Item Selection Bias >>"
        # ">>State Logic Queue Reference >>"
        # ">>Action states Queue Reference >>"
        # ">>True Stop Next State >>"
        # ">>State Logic  >>"
        # ">>> IR Sensors >>>"
        # ">>> Line Sensor Cluster>>>"
        # ">>> Line Sensor Cluster>>>"
        # ">>> Motor control cluster >>>"
        # ">>> yStepper command>>>"
        # ">>> Motor control cluster >>>"
        # ">>> yStepper command>>>"
        # ">>> Motor control cluster >>>"
        # ">>> IR Sensors >>>"
        # ">>> IR Sensors >>>"
        # ">>> yStepper command>>>"
        # ">>> Time cluster >>>"
        # ">>> Yaw >>>"
        # ">>> Stepper position >>>"
        # ">>> Encoders >>>"
        # ">>> Object detection >>>"
        # ">>> Ultrasonic Sensors Detect >>>"
        # ">>> Time cluster >>>"
        # ">>> Yaw >>>"
        # ">>> Stepper position >>>"
        # ">>> Encoders >>>"
        # ">>> Object detection >>>"
        # ">>> Ultrasonic Sensors Detect >>>"
      }
      frame True {
        # ">>State Logic Queue Reference >>"
        # ">>> Box Colour Detection >>>"
        # ">> Item Selection Bias >>"
        # ">>> IR Sensors >>>"
        # ">>> Line Sensor Cluster>>>"
        # ">>> Line Sensor Cluster>>>"
        # ">>> Motor control cluster >>>"
        # ">>> yStepper command>>>"
        # ">>> IR Sensors >>>"
        # ">>> Motor control cluster >>>"
        # ">>State Logic Queue Reference >>"
        # ">>Timeout>>"
        # ">>> yStepper command>>>"
        # ">>> Time cluster >>>"
        # ">>> Object detection >>>"
        # ">>> Yaw >>>"
        # ">>> Ultrasonic Sensors Detect >>>"
        # ">>> Encoders >>>"
        # ">>> Stepper position >>>"
        # ">>State Logic  >>"
        # ">>True Stop Next State >>"
        # ">>Action Queue>>"
        # ">> Manual override >>"
        # ">>> Time cluster >>>"
        # ">>> Yaw >>>"
        # ">>> Stepper position >>>"
        # ">>> Encoders >>>"
        # ">>> Object detection >>>"
        # ">>> Ultrasonic Sensors Detect >>>"
        # ">>Action Queue>>"
        # ">>State Logic Queue Reference >>"
        n191 = Or(x=w319, y=w320) -> (x .or. y?=w318:bool)
        n192 = Unbundle By Name(w299) -> ("Left IR Sensor"=w300:dbl, "Arm IR Sensor"=w296:dbl, "Bottom IR Sensor"=w291:dbl)
        n193 = Unbundle By Name(w294) -> ("Line Detected?"=w295:bool)
        n194 = Unbundle By Name(w305) -> ("Time up flag"=w306:bool)
        n195 = Unbundle By Name(w307) -> ("Yaw"=w308:dbl, "Compass"=w302:dbl)
        n196 = Unbundle By Name(w309) -> ("y Stepper Position"=w311:u8, "z Stepper Position"=w310:u8)
        n197 = Unbundle By Name(w325) -> ("xDistance"=w322:dbl, "yDistance"=w323:dbl, "wDistance"=w324:dbl)
        n198 = Unbundle By Name(w313) -> ("Recognized Object"=w312:bool, "Object X coordinate"=w315:dbl, "Object Y coordinate"=w314:dbl)
        n199 = Unbundle By Name(w336) -> ("PING_A"=w328:u8, "PING_B"=w327:u8, "PING_C"=w326:u8, "PING_D"=w321:u8)
        n200 = case shown="43" w335 {
          tunnel: [w341 w353 w367 w378 w496 w513 w559 w596 w651 w693 w741 w785 w840 w888 w932 w992 w1033 w1076 w1125 w1168 w1221 w1259 w1311 w1355 w1399 w1429 w1447 w1493 w1534 w1583 w1636 w1675 w1724 w1767 w1820 w1858 w1910 w1946 w1995 w2038 w2089 w2133 w2178 w2228 w2269 w2317 w2356 w2398 w2453 w2507 w2545 w2591 w2640 w2681 w2725] -> w334
          tunnel: w333 -> [w341 w356 w368 w381 w498 w514 w560 w605 w649 w697 w742 w791 w833 w891 w939 w982 w1036 w1082 w1124 w1171 w1211 w1265 w1301 w1350 w1390 w1429 w1437 w1496 w1540 w1582 w1635 w1681 w1723 w1770 w1810 w1864 w1900 w1950 w2002 w2043 w2094 w2138 w2182 w2226 w2270 w2318 w2358 w2408 w2463 w2506 w2549 w2597 w2639 w2685 w2729]
          tunnel: [State_Type_Definitions,_for_0.26g_versions_and_later_2."Idle" ("Enum") State_Type_Definitions,_for_0.26g_versions_and_later_2."Idle" ("Enum") w363 w380 State_Type_Definitions,_for_0.26g_versions_and_later_2."Shutdown" ("Enum") w515 w561 w603 w652 w694 w740 w786 w839 w889 w934 w991 w1034 w1083 w1126 w1170 w1220 w1266 w1310 w1356 w1391 State_Type_Definitions,_for_0.26g_versions_and_later_2."Idle" ("Enum") w1446 w1494 w1541 w1584 w1637 w1682 w1725 w1769 w1819 w1865 w1909 w1947 w1996 w2039 w2090 w2134 w2179 w2229 w2268 w2316 w2357 w2403 w2464 w2508 w2546 w2592 w2641 w2682 w2726] -> w332
          tunnel: w331 -> [_ _ w366 w384 _ w519 w566 w599 w648 w698 w749 w790 w837 w892 w938 w989 w1031 w1081 w1122 w1172 w1218 w1264 w1308 w1353 w1398 _ w1444 w1491 w1539 w1580 w1633 w1680 w1721 w1771 w1817 w1863 w1907 w1954 w2001 w2046 w2097 w2141 w2185 w2225 w2271 w2311 w2359 w2407 w2462 w2505 w2553 w2596 w2638 w2689 w2730]
          tunnel: w330 -> [_ _ _ w383 _ w518 w565 w598 w647 w699 w748 w789 w836 w885 w937 w988 w1030 w1080 w1121 w1173 w1217 w1263 w1307 w1352 w1396 _ w1443 w1490 w1538 w1579 w1632 w1679 w1720 w1772 w1816 w1862 w1906 w1949 w2000 w2045 w2096 w2140 w2181 w2224 w2272 w2312 w2360 w2406 w2461 w2504 w2552 w2595 w2637 w2688 w2731]
          tunnel: w329 -> [_ _ w365 w379 _ w517 w564 w597 w646 w700 w747 w788 w835 w884 w936 w990 w1032 w1079 w1120 w1174 w1219 w1262 w1309 w1351 w1397 _ w1445 w1492 w1537 w1578 w1631 w1678 w1719 w1773 w1818 w1861 w1908 w1953 w1999 w2044 w2095 w2139 w2184 w2223 w2273 w2313 w2361 w2405 w2460 w2503 w2551 w2594 w2636 w2687 w2732]
          tunnel: w318 -> [_ _ _ _ _ w504 w558 w604 w645 w701 w744 w784 w838 w890 w940 w983 w1037 w1077 w1123 w1175 w1212 w1260 w1302 w1354 w1394 _ w1438 w1497 w1535 w1581 w1634 w1676 w1722 w1774 w1811 w1859 w1901 w1952 w1994 w2042 w2093 w2137 w2183 w2222 w2274 w2314 w2362 w2404 w2459 w2502 w2550 w2593 w2635 w2686 w2733]
          tunnel: w328 -> [_ _ _ _ _ _ _ _ _ _ _ _ _ _ _ _ _ _ _ _ _ _ _ _ _ _ _ _ _ _ _ _ _ _ _ _ _ _ _ _ _ _ _ _ _ _ _ _ _ _ _ _ _ _ _]
          tunnel: w327 -> [_ _ _ _ _ _ _ _ w644 _ _ _ w829 w873 w930 _ _ _ _ _ _ _ _ _ _ _ _ w1483 _ _ _ _ _ _ _ _ _ _ _ _ _ _ _ _ _ _ _ _ w2457 _ _ _ _ _ _]
          tunnel: w326 -> [_ _ _ _ _ _ _ _ w643 _ _ _ w830 w874 w931 _ _ _ _ _ _ _ _ _ _ _ _ w1484 _ _ _ _ _ _ _ _ _ _ _ _ _ _ _ _ _ _ _ _ w2458 _ _ _ _ _ _]
          tunnel: w324 -> [_ _ _ _ _ _ _ _ _ _ w746 _ _ _ _ _ _ _ _ _ _ _ _ _ _ _ _ _ _ _ _ _ _ _ _ _ _ _ _ _ _ _ _ _ _ _ _ w2401 _ _ _ _ _ _ _]
          tunnel: w323 -> [_ _ _ _ _ w512 w557 _ _ w692 _ _ _ _ w935 _ _ _ _ _ _ _ _ _ _ _ _ _ _ _ _ _ _ _ _ _ _ _ _ _ _ _ _ _ _ _ _ _ w2449 _ _ _ _ _ _]
          tunnel: w322 -> [_ _ _ _ _ _ _ _ _ _ _ _ _ w879 _ _ _ _ _ _ _ _ _ _ _ _ _ _ _ _ w1622 _ _ _ _ _ _ _ _ _ _ _ _ _ w2263 _ _ _ _ _ _ _ w2634 _ _]
          tunnel: w321 -> [_ _ _ _ _ _ _ _ _ _ _ _ _ _ _ _ _ _ _ _ _ _ _ _ _ _ _ _ _ _ _ _ _ _ _ _ _ _ _ _ _ _ _ _ _ _ _ _ _ _ _ _ _ _ _]
          tunnel: [State_Type_Definitions,_for_0.26g_versions_and_later_2."Idle" ("Enum") State_Type_Definitions,_for_0.26g_versions_and_later_2."Idle" ("Enum") State_Type_Definitions,_for_0.26g_versions_and_later_2."Idle" ("Enum") State_Type_Definitions,_for_0.26g_versions_and_later_2."Idle" ("Enum") State_Type_Definitions,_for_0.26g_versions_and_later_2."Shutdown" ("Enum") w510 w555 w602 w650 w695 w737 w783 w832 w887 w933 w993 w1035 w1075 w1127 w1169 w1222 w1258 w1312 w1357 w1392 w1431 w1448 w1495 w1533 w1585 w1638 w1674 w1726 w1768 w1821 w1857 w1911 w1948 w1997 w2041 w2092 w2136 w2180 w2227 w2267 w2315 w2355 w2402 w2465 w2509 w2547 w2590 w2642 w2683 w2727] -> w317
          tunnel: w316 -> [_ _ w363 _ _ _ _ _ _ _ _ _ _ _ _ _ _ _ _ _ _ _ _ _ _ w1431 _ _ _ _ _ _ _ _ _ _ _ _ _ _ _ _ _ _ _ _ _ _ _ _ _ _ _ _ _]
          tunnel: w312 -> [_ _ _ _ _ _ _ _ _ _ _ _ _ _ _ _ _ _ _ _ _ _ _ _ w1393 _ _ _ _ _ _ _ _ _ _ _ _ _ _ _ _ _ _ _ _ _ _ _ _ _ _ _ _ _ _]
          tunnel: w315 -> [_ _ _ _ _ _ _ _ _ _ _ _ _ _ _ _ _ _ _ _ _ _ _ _ _ _ _ _ _ _ w1628 _ _ _ _ _ _ _ _ _ _ _ _ _ _ _ _ _ _ _ _ _ _ _ _]
          tunnel: w314 -> [_ _ _ _ _ _ _ _ _ _ _ _ _ _ _ _ _ _ _ w1164 _ _ _ _ _ _ _ _ _ _ _ _ _ w1763 _ _ _ _ _ _ _ _ _ _ _ _ _ _ _ _ _ _ _ _ _]
          tunnel: w311 -> [_ _ _ _ _ _ _ _ _ _ _ _ _ _ _ _ _ _ _ w1163 _ _ _ _ _ _ _ _ _ _ _ _ _ w1762 _ _ _ _ _ _ _ _ _ _ _ _ _ _ _ _ _ _ _ _ _]
          tunnel: w310 -> [_ _ _ _ _ _ _ w601 _ _ _ w781 _ _ _ w986 _ w1071 _ _ w1215 _ w1305 w1349 _ _ w1441 _ _ _ _ _ _ _ w1814 _ w1904 w1951 _ _ _ _ _ _ _ _ _ _ _ _ _ _ _ _ _]
          tunnel: w308 -> [_ _ _ _ _ _ _ _ _ _ _ _ _ _ _ _ _ _ _ _ _ _ _ _ _ _ _ _ _ _ _ _ _ _ _ _ _ _ _ _ _ _ _ _ _ _ _ _ _ _ _ _ _ _ _]
          tunnel: w306 -> [_ _ _ _ _ _ _ _ _ _ _ _ _ _ _ _ w1025 _ w1117 _ _ w1256 _ _ _ _ _ _ w1531 w1575 _ w1672 w1716 _ _ w1855 _ _ _ _ _ _ w2174 w2218 _ w2310 w2354 _ _ _ w2548 w2589 _ w2684 w2728]
          tunnel: w304 -> [w339 w351 w362 w376 w494 w509 w554 w600 w642 w696 w736 w782 w831 w883 w929 w981 w1028 w1074 w1118 w1166 w1210 w1257 w1300 w1346 w1389 w1432 w1436 w1488 w1532 w1576 w1629 w1673 w1717 w1765 w1809 w1856 w1899 w1945 w1998 w2040 w2091 w2135 w2177 w2221 w2276 w2320 w2364 w2410 w2467 w2511 w2555 w2599 w2647 w2691 w2735]
          tunnel: [w339 w350 w362 w376 w494 w509 w554 w600 w642 w696 w736 w782 w831 w883 w929 w981 w1028 w1074 w1118 w1165 w1210 w1257 w1300 w1346 w1389 w1432 w1436 w1488 w1532 w1576 w1629 w1673 w1717 w1764 w1809 w1856 w1899 w1945 w1998 w2040 w2091 w2135 w2177 w2221 w2276 w2320 w2364 w2410 w2467 w2511 w2555 w2599 w2647 w2691 w2735] -> w303
          tunnel: w302 -> [_ _ _ _ _ _ _ _ _ _ _ _ _ _ _ _ _ _ _ _ _ _ _ _ _ _ _ _ _ _ _ _ _ _ _ _ _ _ w1993 _ _ _ _ _ _ _ _ _ _ _ _ _ _ _ _]
          tunnel: [_ _ _ TRUE _ _ _ _ _ _ _ _ _ _ _ _ _ _ _ _ _ _ _ _ _ _ _ _ _ _ _ _ _ _ _ _ _ _ _ _ _ _ _ _ _ _ _ _ _ _ _ _ _ _ _] -> w301
          tunnel: w300 -> [_ _ _ _ _ _ _ _ _ _ _ _ _ _ _ _ _ _ _ _ _ _ _ _ _ _ _ _ _ _ _ _ _ _ _ _ _ _ _ _ _ _ _ _ _ _ _ _ _ _ _ _ _ _ _]
          tunnel: w298 -> [w338 w348 w361 w374 w493 w508 w553 w595 w641 w689 w735 w778 w824 w872 w928 w980 w1027 w1073 w1116 w1160 w1209 w1255 w1299 w1345 w1388 w1433 w1435 w1481 w1530 w1574 w1625 w1671 w1715 w1759 w1808 w1854 w1898 w1944 w1989 w2037 w2088 w2132 w2176 w2220 w2278 w2322 w2366 w2412 w2469 w2513 w2557 w2601 w2649 w2693 w2737]
          tunnel: [w338 w347 w361 w374 w493 w508 w553 w595 w641 w689 w735 w778 w824 w872 w928 w980 w1027 w1073 w1116 w1160 w1209 w1255 w1299 w1345 w1388 w1433 w1435 w1481 w1530 w1574 w1624 w1671 w1715 w1759 w1808 w1854 w1898 w1944 w1989 w2037 w2088 w2132 w2176 w2220 w2278 w2322 w2366 w2412 w2469 w2513 w2557 w2601 w2649 w2693 w2737] -> w297